vi "FlexMag - 23-03-2023.vi"() -> ()   [LabVIEW 2018] (continued)
                  }
                  frame #1 {
                    n264 = Wait (ms)(milliseconds to wait=u32 500) -> ()  [unwired: 1 out]
                  }
                  frame #2 {
                    n265 = local write "CH3_MP_DO"(TRUE ("CH3_MP_DO")) -> ()
                  }
                }
              }
            }
          }
        }
        n266 = case shown="True" w560 {
          tunnel: "mp3 stop safety" -> [_ w668]
          frame False {
          }
          frame True {
            n267 = case shown="True" w668 {
              frame False {
                n268 = local write "Warning Message"("CH3 MP Cannot be stopped !" ("Warning Message")) -> ()
              }
              frame True {
                n269 = stacked-sequence {
                  frame #0 {
                    w670 = FALSE ("CH3_MP_DO")
                    n270 = local write "CH3_MP_DO"(w670) -> ()
                    n271 = local write "CH3_PL_ATM_DO"(w670) -> ()
                    n272 = local write "CH3_CH_ATM_DO"(w670) -> ()
                  }
                  frame #1 {
                    n273 = Wait (ms)(milliseconds to wait=u32 500) -> ()  [unwired: 1 out]
                  }
                  frame #2 {
                    n274 = local write "CH3_PL_VBV_DO"(TRUE ("CH3_PL_VBV_DO")) -> ()
                  }
                }
              }
            }
          }
        }
        n275 = case shown="True" w562 {
          tunnel: "mp4 start safety" -> [_ w663]
          frame False {
          }
          frame True {
            n276 = case shown="True" w663 {
              frame False {
                n277 = local write "Warning Message"("CH4 MP Cannot be started !" ("Warning Message")) -> ()
              }
              frame True {
                n278 = stacked-sequence {
                  frame #0 {
                    w665 = TRUE ("CH1_PL_ATM_DO")
                    n279 = local write "CH4_PL_ATM_DO"(w665) -> ()
                    n280 = local write "CH4_CH_ATM_DO"(w665) -> ()
                  }
                  frame #1 {
                    n281 = Wait (ms)(milliseconds to wait=u32 500) -> ()  [unwired: 1 out]
                  }
                  frame #2 {
                    n282 = local write "CH4_MP_DO"(TRUE ("CH4_MP_DO")) -> ()
                  }
                }
              }
            }
          }
        }
        n283 = case shown="True" w561 {
          tunnel: "mp4 stop safety" -> [_ w658]
          frame False {
          }
          frame True {
            n284 = case shown="True" w658 {
              frame False {
                n285 = local write "Warning Message"("CH4 MP Cannot be stopped !" ("Warning Message")) -> ()
              }
              frame True {
                n286 = stacked-sequence {
                  frame #0 {
                    w660 = FALSE ("CH4_MP_DO")
                    n287 = local write "CH4_MP_DO"(w660) -> ()
                    n288 = local write "CH4_PL_ATM_DO"(w660) -> ()
                    n289 = local write "CH4_CH_ATM_DO"(w660) -> ()
                  }
                  frame #1 {
                    n290 = Wait (ms)(milliseconds to wait=u32 500) -> ()  [unwired: 1 out]
                  }
                  frame #2 {
                    n291 = local write "CH4_PL_VBV_DO"(TRUE ("CH4_PL_VBV_DO")) -> ()
                  }
                }
              }
            }
          }
        }
        n292 = case shown="True" w503 {
          tunnel: "tpbv1 open safety" -> [_ w640]
          frame False {
          }
          frame True {
            n293 = case shown="True" w640 {
              frame False {
                n294 = local write "Warning Message"("CH1 TP BV Cannot be opened !" ("Warning Message")) -> ()
              }
              frame True {
                n295 = local write "CH1_TP_BV_DO"(TRUE ("CH1_MP_DO")) -> ()
              }
            }
          }
        }
        n296 = case shown="True" w504 {
          tunnel: "tpbv1 close safety" -> [_ w637]
          frame False {
          }
          frame True {
            n297 = case shown="True" w637 {
              frame False {
                n298 = local write "Warning Message"("CH1 TP BV Cannot be closed !" ("Warning Message")) -> ()
              }
              frame True {
                n299 = local write "CH1_TP_BV_DO"(FALSE ("CH1_MP_DO")) -> ()
              }
            }
          }
        }
        n300 = case shown="True" w506 {
          tunnel: "tpbv2 open safety" -> [_ w634]
          frame False {
          }
          frame True {
            n301 = case shown="True" w634 {
              frame False {
                n302 = local write "Warning Message"("CH2 TP BV Cannot be opened !" ("Warning Message")) -> ()
              }
              frame True {
                n303 = local write "CH2_TP_BV_DO"(TRUE ("CH2_MP_DO")) -> ()
              }
            }
          }
        }
        n304 = case shown="True" w505 {
          tunnel: "tpbv2 close safety" -> [_ w631]
          frame False {
          }
          frame True {
            n305 = case shown="True" w631 {
              frame False {
                n306 = local write "Warning Message"("CH2 TP BV Cannot be closed !" ("Warning Message")) -> ()
              }
              frame True {
                n307 = local write "CH2_TP_BV_DO"(FALSE ("CH2_MP_DO")) -> ()
              }
            }
          }
        }
        n308 = case shown="True" w510 {
          tunnel: "tpbv3 open safety" -> [_ w628]
          frame False {
          }
          frame True {
            n309 = case shown="True" w628 {
              frame False {
                n310 = local write "Warning Message"("CH3 TP BV Cannot be opened !" ("Warning Message")) -> ()
              }
              frame True {
                n311 = local write "CH3_TP_BV_DO"(TRUE ("CH3_MP_DO")) -> ()
              }
            }
          }
        }
        n312 = case shown="True" w509 {
          tunnel: "tpbv3 close safety" -> [_ w625]
          frame False {
          }
          frame True {
            n313 = case shown="True" w625 {
              frame False {
                n314 = local write "Warning Message"("CH3 TP BV Cannot be closed !" ("Warning Message")) -> ()
              }
              frame True {
                n315 = local write "CH3_TP_BV_DO"(FALSE ("CH3_MP_DO")) -> ()
              }
            }
          }
        }
        n316 = case shown="True" w507 {
          tunnel: "tpbv4 open safety" -> [_ w622]
          frame False {
          }
          frame True {
            n317 = case shown="True" w622 {
              frame False {
                n318 = local write "Warning Message"("CH4 TP BV Cannot be opened !" ("Warning Message")) -> ()
              }
              frame True {
                n319 = local write "CH4_TP_BV_DO"(TRUE ("CH4_MP_DO")) -> ()
              }
            }
          }
        }
        n320 = case shown="True" w508 {
          tunnel: "tpbv4 close safety" -> [_ w619]
          frame False {
          }
          frame True {
            n321 = case shown="True" w619 {
              frame False {
                n322 = local write "Warning Message"("CH4 TP BV Cannot be closed !" ("Warning Message")) -> ()
              }
              frame True {
                n323 = local write "CH4_TP_BV_DO"(FALSE ("CH4_MP_DO")) -> ()
              }
            }
          }
        }
        n324 = Or(x="plvbv1 open gui", y="plvbv1 open gui 1") -> (x .or. y?=w511:bool)
        n325 = Or(x="plvbv2 open gui", y="plvbv2 open gui 1") -> (x .or. y?=w516:bool)
        n326 = Or(x="plvbv3 open gui", y="plvbv3 open gui 1") -> (x .or. y?=w522:bool)
        n327 = Or(x="plvbv4 open gui", y="plvbv4 open gui 1") -> (x .or. y?=w519:bool)
        n328 = Or(x="chvbv1 open gui", y="chvbv1 open gui 1") -> (x .or. y?=w478:bool)
        n329 = Or(x="chvbv2 open gui", y="chvbv2 open gui 1") -> (x .or. y?=w475:bool)
        n330 = Or(x="chvbv3 open gui", y="chvbv3 open gui 1") -> (x .or. y?=w471:bool)
        n331 = Or(x="chvbv4 open gui", y="chvbv4 open gui 1") -> (x .or. y?=w474:bool)
        n332 = Or(x="plvbv1 close gui", y="plvbv1 close gui 1") -> (x .or. y?=w513:bool)
        n333 = Or(x="plvbv2 close gui", y="plvbv2 close gui 1") -> (x .or. y?=w515:bool)
        n334 = Or(x="plvbv3 close gui", y="plvbv3 close gui 1") -> (x .or. y?=w521:bool)
        n335 = Or(x="plvbv4 close gui", y="plvbv4 close gui 1") -> (x .or. y?=w520:bool)
        n336 = Or(x="chvbv1 close gui", y="chvbv1 close gui 1") -> (x .or. y?=w477:bool)
        n337 = Or(x="chvbv2 close gui", y="chvbv2 close gui 1") -> (x .or. y?=w476:bool)
        n338 = Or(x="chvbv3 close gui", y="chvbv3 close gui 1") -> (x .or. y?=w472:bool)
        n339 = Or(x="chvbv4 close gui", y="chvbv4 close gui 1") -> (x .or. y?=w473:bool)
        n340 = Compound Arithmetic op=OR("bgbv1 open gui 2", "bgbv1 open gui", "bgbv1 open gui 3") -> (w440:bool)
        n341 = Compound Arithmetic op=OR("bgbv2 open gui 2", "bgbv2 open gui", "bgbv1 open gui 1") -> (w443:bool)
        n342 = Compound Arithmetic op=OR("bgbv3 open gui 2", "bgbv3 open gui", "bgbv3 open gui 1") -> (w447:bool)
        n343 = Compound Arithmetic op=OR("bgbv4 open gui 2", "bgbv4 open gui", "bgbv4 open gui 1") -> (w444:bool)
        n344 = Compound Arithmetic op=OR("bgbv1 close gui 2", "bgbv1 close gui", "bgbv1 close gui 1") -> (w441:bool)
        n345 = Compound Arithmetic op=OR("bgbv2 close gui 2", "bgbv2 close gui", "bgbv2 close gui 1") -> (w442:bool)
        n346 = Compound Arithmetic op=OR("bgbv3 close gui 2", "bgbv3 close gui", "bgbv3 close gui 1") -> (w446:bool)
        n347 = Compound Arithmetic op=OR("bgbv4 close gui 2", "bgbv4 close gui", "bgbv4 close gui 1") -> (w445:bool)
        n348 = case shown="True" w511 {
          tunnel: "plvbv1 open safety" -> [_ w656]
          frame False {
          }
          frame True {
            n349 = case shown="True" w656 {
              frame False {
                n350 = local write "Warning Message"("CH1 PL VBV Cannot be opened !" ("Warning Message")) -> ()
              }
              frame True {
              }
            }
          }
        }
        n351 = case shown="True" w513 {
          frame False {
          }
          frame True {
            n352 = local write "CH1_PL_VBV_DO"(FALSE ("CH1_PL_VBV_DO")) -> ()
          }
        }
        n353 = case shown="True" w516 {
          tunnel: "plvbv2 open safety" -> [_ w652]
          frame False {
          }
          frame True {
            n354 = case shown="True" w652 {
              frame False {
                n355 = local write "Warning Message"("CH2 PL VBV Cannot be opened !" ("Warning Message")) -> ()
              }
              frame True {
                n356 = local write "CH2_PL_VBV_DO"(TRUE ("CH2_PL_VBV_DO")) -> ()
              }
            }
          }
        }
        n357 = case shown="True" w515 {
          frame False {
          }
          frame True {
            n358 = local write "CH2_PL_VBV_DO"(FALSE ("CH2_PL_VBV_DO")) -> ()
          }
        }
        n359 = case shown="True" w522 {
          tunnel: "plvbv3 open safety" -> [_ w648]
          frame False {
          }
          frame True {
            n360 = case shown="True" w648 {
              frame False {
                n361 = local write "Warning Message"("CH3 PL VBV Cannot be opened !" ("Warning Message")) -> ()
              }
              frame True {
                n362 = local write "CH3_PL_VBV_DO"(TRUE ("CH3_PL_VBV_DO")) -> ()
              }
            }
          }
        }
        n363 = case shown="True" w521 {
          frame False {
          }
          frame True {
            n364 = local write "CH3_PL_VBV_DO"(FALSE ("CH3_PL_VBV_DO")) -> ()
          }
        }
        n365 = case shown="True" w519 {
          tunnel: "plvbv4 open safety" -> [_ w644]
          frame False {
          }
          frame True {
            n366 = case shown="True" w644 {
              frame False {
                n367 = local write "Warning Message"("CH4 PL VBV Cannot be opened !" ("Warning Message")) -> ()
              }
              frame True {
                n368 = local write "CH4_PL_VBV_DO"(TRUE ("CH4_PL_VBV_DO")) -> ()
              }
            }
          }
        }
        n369 = case shown="True" w520 {
          frame False {
          }
          frame True {
            n370 = local write "CH4_PL_VBV_DO"(FALSE ("CH4_PL_VBV_DO")) -> ()
          }
        }
        n371 = case shown="True" w440 {
          tunnel: "bgbv1 open safety" -> [_ w600]
          frame False {
          }
          frame True {
            n372 = case shown="True" w600 {
              frame False {
                n373 = local write "Warning Message"("CH1 BG BV Cannot be opened !" ("Warning Message")) -> ()
              }
              frame True {
                n374 = local write "CH1_BG_BV_DO"(TRUE ("CH1_MP_DO")) -> ()
              }
            }
          }
        }
        n375 = case shown="True" w441 {
          frame False {
          }
          frame True {
            n376 = local write "CH1_BG_BV_DO"(FALSE ("CH1_MP_DO")) -> ()
          }
        }
        n377 = case shown="True" w443 {
          tunnel: "bgbv2 open safety" -> [_ w596]
          frame False {
          }
          frame True {
            n378 = case shown="True" w596 {
              frame False {
                n379 = local write "Warning Message"("CH2 BG BV Cannot be opened !" ("Warning Message")) -> ()
              }
              frame True {
                n380 = local write "CH2_BG_BV_DO"(TRUE ("CH2_MP_DO")) -> ()
              }
            }
          }
        }
        n381 = case shown="True" w442 {
          frame False {
          }
          frame True {
            n382 = local write "CH2_BG_BV_DO"(FALSE ("CH2_MP_DO")) -> ()
          }
        }
        n383 = case shown="True" w447 {
          tunnel: "bgbv3 open safety" -> [_ w592]
          frame False {
          }
          frame True {
            n384 = case shown="True" w592 {
              frame False {
                n385 = local write "Warning Message"("CH3 BG BV Cannot be opened !" ("Warning Message")) -> ()
              }
              frame True {
                n386 = local write "CH3_BG_BV_DO"(TRUE ("CH3_MP_DO")) -> ()
              }
            }
          }
        }
        n387 = case shown="True" w446 {
          frame False {
          }
          frame True {
            n388 = local write "CH3_BG_BV_DO"(FALSE ("CH3_MP_DO")) -> ()
          }
        }
        n389 = case shown="True" w444 {
          tunnel: "bgbv4 open safety" -> [_ w588]
          frame False {
          }
          frame True {
            n390 = case shown="True" w588 {
              frame False {
                n391 = local write "Warning Message"("CH4 BG BV Cannot be opened !" ("Warning Message")) -> ()
              }
              frame True {
                n392 = local write "CH4_BG_BV_DO"(TRUE ("CH4_MP_DO")) -> ()
              }
            }
          }
        }
        n393 = case shown="True" w445 {
          frame False {
          }
          frame True {
            n394 = local write "CH4_BG_BV_DO"(FALSE ("CH4_MP_DO")) -> ()
          }
        }
        n395 = case shown="True" w478 {
          tunnel: "chvbv1 open safety" -> [_ w616]
          frame False {
          }
          frame True {
            n396 = case shown="True" w616 {
              frame False {
                n397 = local write "Warning Message"("CH1 VBV Cannot be opened !" ("Warning Message")) -> ()
              }
              frame True {
                n398 = local write "CH1_CH_VBV_DO"(TRUE ("CH1_MP_DO")) -> ()
              }
            }
          }
        }
        n399 = case shown="True" w477 {
          frame False {
          }
          frame True {
            n400 = local write "CH1_CH_VBV_DO"(FALSE ("CH1_MP_DO")) -> ()
          }
        }
        n401 = case shown="True" w475 {
          tunnel: "chvbv2 open safety" -> [_ w612]
          frame False {
          }
          frame True {
            n402 = case shown="True" w612 {
              frame False {
                n403 = local write "Warning Message"("CH2 VBV Cannot be opened !" ("Warning Message")) -> ()
              }
              frame True {
                n404 = local write "CH2_CH_VBV_DO"(TRUE ("CH2_MP_DO")) -> ()
              }
            }
          }
        }
        n405 = case shown="True" w476 {
          frame False {
          }
          frame True {
            n406 = local write "CH2_CH_VBV_DO"(FALSE ("CH2_MP_DO")) -> ()
          }
        }
        n407 = case shown="True" w471 {
          tunnel: "chvbv3 open safety" -> [_ w608]
          frame False {
          }
          frame True {
            n408 = case shown="True" w608 {
              frame False {
                n409 = local write "Warning Message"("CH3 VBV Cannot be opened !" ("Warning Message")) -> ()
              }
              frame True {
                n410 = local write "CH3_CH_VBV_DO"(TRUE ("CH3_MP_DO")) -> ()
              }
            }
          }
        }
        n411 = case shown="True" w472 {
          frame False {
          }
          frame True {
            n412 = local write "CH3_CH_VBV_DO"(FALSE ("CH3_MP_DO")) -> ()
          }
        }
        n413 = case shown="True" w474 {
          tunnel: "chvbv4 open safety" -> [_ w604]
          frame False {
          }
          frame True {
            n414 = case shown="True" w604 {
              frame False {
                n415 = local write "Warning Message"("CH4 VBV Cannot be opened !" ("Warning Message")) -> ()
              }
              frame True {
                n416 = local write "CH4_CH_VBV_DO"(TRUE ("CH4_MP_DO")) -> ()
              }
            }
          }
        }
        n417 = case shown="True" w473 {
          frame False {
          }
          frame True {
            n418 = local write "CH4_CH_VBV_DO"(FALSE ("CH4_MP_DO")) -> ()
          }
        }
      }
      frame #1 {
        n419 = Or(x="ch1 trnsbp left open gui", y="ch1 trnsbp left open gui1") -> (x .or. y?=w791:bool)
        n420 = Or(x="ch2 trnsbp right open gui", y="ch2 trnsbp right open gui 1") -> (x .or. y?=w788:bool)
        n421 = Or(x="sov3 open gui", y="sov3 open gui 2") -> (x .or. y?=w801:bool)
        n422 = Or(x="ch2 trnsbp left open gui", y="ch2 trnsbp left open gui 1") -> (x .or. y?=w781:bool)
        n423 = Or(x="ch1 trnsbp left close gui", y="ch1 trnsbp left close gui 1") -> (x .or. y?=w793:bool)
        n424 = Or(x="ch2 trnsbp right close gui", y="ch2 trnsbp right close gui 1") -> (x .or. y?=w787:bool)
        n425 = Or(x="ch3 trnsbp right open gui", y="ch3 trnsbp right open gui 1") -> (x .or. y?=w775:bool)
        n426 = Or(x="sov1 open gui", y="sov1 open gui 2") -> (x .or. y?=w823:bool)
        n427 = Or(x="sov3 close gui", y="sov3 close gui 2") -> (x .or. y?=w802:bool)
        n428 = Or(x="ch2 trnsbp left close gui", y="ch2 trnsbp left close gui 1") -> (x .or. y?=w782:bool)
        n429 = Or(x="ch3 trnsbp left open gui", y="ch3 trnsbp left open gui 1") -> (x .or. y?=w767:bool)
        n430 = Or(x="ch4 trnsbp right open gui", y="ch4 trnsbp right open gui 1") -> (x .or. y?=w762:bool)
        n431 = Or(x="ch3 trnsbp right close gui", y="ch3 trnsbp right close gui 1") -> (x .or. y?=w774:bool)
        n432 = Or(x="sov1 close gui", y="sov1 close gui 2") -> (x .or. y?=w820:bool)
        n433 = Or(x="ch3 trnsbp left close gui", y="ch3 trnsbp left close gui 1") -> (x .or. y?=w768:bool)
        n434 = Or(x="ch4 trnsbp right close gui", y="ch4 trnsbp right close gui 1") -> (x .or. y?=w761:bool)
        n435 = case shown="True" w788 {
          tunnel: "ch2 trnsbp right open safety" -> [_ w908]
          frame False {
          }
          frame True {
            n436 = case shown="True" w908 {
              frame False {
                n437 = local write "Warning Message"("CH2 TRNS BP Right Cannot be opened !" ("Warning Message")) -> ()
              }
              frame True {
                n438 = local write "CH2_Trns_BP_Right_DO"(TRUE ("CH4_MP_DO")) -> ()
              }
            }
          }
        }
        n439 = case shown="True" w781 {
          tunnel: "ch2 trnsbp left open safety" -> [_ w904]
          frame False {
          }
          frame True {
            n440 = case shown="True" w904 {
              frame False {
                n441 = local write "Warning Message"("CH2 TRNS BP Left Cannot be opened !" ("Warning Message")) -> ()
              }
              frame True {
                n442 = local write "CH2_Trns_BP_Left_DO"(TRUE ("CH4_MP_DO")) -> ()
              }
            }
          }
        }
        n443 = case shown="True" w793 {
          frame False {
          }
          frame True {
            n444 = local write "CH1_Trns_BP_Left_DO"(FALSE ("CH4_MP_DO")) -> ()
          }
        }
        n445 = case shown="True" w787 {
          frame False {
          }
          frame True {
            n446 = local write "CH2_Trns_BP_Right_DO"(FALSE ("CH4_MP_DO")) -> ()
          }
        }
        n447 = case shown="True" w775 {
          tunnel: "ch3 trnsbp right open safety" -> [_ w900]
          frame False {
          }
          frame True {
            n448 = case shown="True" w900 {
              frame False {
                n449 = local write "Warning Message"("CH3 TRNS BP Right Cannot be opened !" ("Warning Message")) -> ()
              }
              frame True {
                n450 = local write "CH3_Trns_BP_Right_DO"(TRUE ("CH4_MP_DO")) -> ()
              }
            }
          }
        }
        n451 = case shown="True" w802 {
          frame False {
          }
          frame True {
            n452 = local write "CH3_SoV_Ar_DO"(FALSE ("CH4_MP_DO")) -> ()
          }
        }
        n453 = case shown="True" w782 {
          frame False {
          }
          frame True {
            n454 = local write "CH2_Trns_BP_Left_DO"(FALSE ("CH4_MP_DO")) -> ()
          }
        }
        n455 = case shown="True" w767 {
          tunnel: "ch3 trnsbp left open safety" -> [_ w896]
          frame False {
          }
          frame True {
            n456 = case shown="True" w896 {
              frame False {
                n457 = local write "Warning Message"("CH3 TRNS BP Left Cannot be opened !" ("Warning Message")) -> ()
              }
              frame True {
                n458 = local write "CH3_Trns_BP_Left_DO"(TRUE ("CH4_MP_DO")) -> ()
              }
            }
          }
        }
        n459 = case shown="True" w762 {
          tunnel: "ch4 trnsbp right open safety" -> [_ w892]
          frame False {
          }
          frame True {
            n460 = case shown="True" w892 {
              frame False {
                n461 = local write "Warning Message"("CH4 TRNS BP Right Cannot be opened !" ("Warning Message")) -> ()
              }
              frame True {
                n462 = local write "CH4_Trns_BP_Right_DO"(TRUE ("CH4_MP_DO")) -> ()
              }
            }
          }
        }
        n463 = case shown="True" "CH1 petcool up" {
          frame False {
          }
          frame True {
            n464 = local write "CH1_PetCool_Down_DO"(FALSE ("CH4_MP_DO")) -> ()
            n465 = local write "CH1_PetCool_Up_DO"(TRUE ("CH4_MP_DO")) -> ()
          }
        }
        n466 = case shown="True" "CH2 petcool up" {
          frame False {
          }
          frame True {
            n467 = local write "CH2_PetCool_Down_DO"(FALSE ("CH4_MP_DO")) -> ()
            n468 = local write "CH2_PetCool_Up_DO"(TRUE ("CH4_MP_DO")) -> ()
          }
        }
        n469 = case shown="True" w791 {
          tunnel: "ch1 trnsbp left open safety" -> [_ w912]
          frame False {
          }
          frame True {
            n470 = case shown="True" w912 {
              frame False {
                n471 = local write "Warning Message"("CH1 TRNS BP Left Cannot be opened !" ("Warning Message")) -> ()
              }
              frame True {
                n472 = local write "CH1_Trns_BP_Left_DO"(TRUE ("CH4_MP_DO")) -> ()
              }
            }
          }
        }
        n473 = case shown="True" w774 {
          frame False {
          }
          frame True {
            n474 = local write "CH3_Trns_BP_Right_DO"(FALSE ("CH4_MP_DO")) -> ()
          }
        }
        n475 = case shown="True" "CH1 petcool down" {
          frame False {
          }
          frame True {
            n476 = local write "CH1_PetCool_Down_DO"(TRUE ("CH4_MP_DO")) -> ()
            n477 = local write "CH1_PetCool_Up_DO"(FALSE ("CH4_MP_DO")) -> ()
          }
        }
        n478 = case shown="True" "CH2 petcool down" {
          frame False {
          }
          frame True {
            n479 = local write "CH2_PetCool_Down_DO"(TRUE ("CH4_MP_DO")) -> ()
            n480 = local write "CH2_PetCool_Up_DO"(FALSE ("CH4_MP_DO")) -> ()
          }
        }
        n481 = case shown="True" w820 {
          frame False {
          }
          frame True {
            n482 = local write "CH1_SoV_Ar_DO"(FALSE ("CH4_MP_DO")) -> ()
          }
        }
        n483 = case shown="True" w801 {
          tunnel: "sov3 open safety" -> [_ w916]
          frame False {
          }
          frame True {
            n484 = case shown="True" w916 {
              frame False {
                n485 = local write "Warning Message"("CH3 SoV Ar Cannot be opened !" ("Warning Message")) -> ()
              }
              frame True {
                n486 = local write "CH3_SoV_Ar_DO"(TRUE ("CH4_MP_DO")) -> ()
              }
            }
          }
        }
        n487 = case shown="True" w768 {
          frame False {
          }
          frame True {
            n488 = local write "CH3_Trns_BP_Left_DO"(FALSE ("CH4_MP_DO")) -> ()
          }
        }
        n489 = case shown="True" w761 {
          frame False {
          }
          frame True {
            n490 = local write "CH4_Trns_BP_Right_DO"(FALSE ("CH4_MP_DO")) -> ()
          }
        }
        n491 = case shown="True" "CH3 petcool up" {
          frame False {
          }
          frame True {
            n492 = local write "CH3_PetCool_Down_DO"(FALSE ("CH4_MP_DO")) -> ()
            n493 = local write "CH3_PetCool_Up_DO"(TRUE ("CH4_MP_DO")) -> ()
          }
        }
        n494 = case shown="True" "CH4 petcool up" {
          frame False {
          }
          frame True {
            n495 = local write "CH4_PetCool_Down_DO"(FALSE ("CH4_MP_DO")) -> ()
            n496 = local write "CH4_PetCool_Up_DO"(TRUE ("CH4_MP_DO")) -> ()
          }
        }
        n497 = case shown="True" "ch3 mag active gui" {
          frame False {
          }
          frame True {
            n498 = local write "DCPS_ SW1 DO"(FALSE ("CH4_MP_DO")) -> ()
            n499 = local write "DCPS_ SW2 DO"(TRUE ("CH4_MP_DO")) -> ()
          }
        }
        n500 = case shown="True" "ch2 mag active gui" {
          frame False {
          }
          frame True {
            n501 = local write "DCPS_ SW1 DO"(TRUE ("CH4_MP_DO")) -> ()
            n502 = local write "DCPS_ SW2 DO"(FALSE ("CH4_MP_DO")) -> ()
          }
        }
        n503 = case shown="True" "CH3 petcool down" {
          frame False {
          }
          frame True {
            n504 = local write "CH3_PetCool_Down_DO"(TRUE ("CH4_MP_DO")) -> ()
            n505 = local write "CH3_PetCool_Up_DO"(FALSE ("CH4_MP_DO")) -> ()
          }
        }
        n506 = case shown="True" "CH4 petcool down" {
          frame False {
          }
          frame True {
            n507 = local write "CH4_PetCool_Down_DO"(TRUE ("CH4_MP_DO")) -> ()
            n508 = local write "CH4_PetCool_Up_DO"(FALSE ("CH4_MP_DO")) -> ()
          }
        }
        n509 = case shown="True" w823 {
          tunnel: "sov1 open safety" -> [_ w928]
          frame False {
          }
          frame True {
            n510 = case shown="True" w928 {
              frame False {
                n511 = local write "Warning Message"("SoV Ar Cannot be opened !" ("Warning Message")) -> ()
              }
              frame True {
                n512 = local write "CH1_SoV_Ar_DO"(TRUE ("CH4_MP_DO")) -> ()
              }
            }
          }
        }
        n513 = Compound Arithmetic op=OR("CH3-4 trns open gui", "CH3-4 trns close gui 1", "CH3-4 trns open gui 2") -> (w733:bool)
        n514 = Compound Arithmetic op=OR("CH3-4 trns close gui", "CH3-4 trns open gui 1", "CH3-4 trns close gui 2") -> (w732:bool)
        n515 = Or(x="sov4 open gui", y="sov4 open gui 2") -> (x .or. y?=w809:bool)
        n516 = Compound Arithmetic op=OR("CH2-3 trns open gui", "CH2-3 trns open gui 1", "CH2-3 trns open gui 2") -> (w743:bool)
        n517 = Compound Arithmetic op=OR("CH1-2 trns open gui", "CH1-2 trns open gui 2", "CH1-2 trns open gui 1") -> (w749:bool)
        n518 = Or(x="sov2 open gui", y="sov2 open gui 2") -> (x .or. y?=w815:bool)
        n519 = Or(x="sov4 close gui", y="sov4 close gui 2") -> (x .or. y?=w808:bool)
        n520 = Compound Arithmetic op=OR("CH2-3 trns close gui", "CH2-3 trns close gui 1", "CH2-3 trns close gui 2") -> (w742:bool)
        n521 = Compound Arithmetic op=OR("CH1-2 trns close gui", "CH1-2 trns close gui 2", "CH1-2 trns close gui 1") -> (w750:bool)
        n522 = Or(x="sov2 close gui", y="sov2 close gui 2") -> (x .or. y?=w816:bool)
        n523 = case shown="True" "CH4 cstfix up" {
          frame False {
          }
          frame True {
            n524 = local write "CH4_Cst_Fix_DO"(FALSE ("CH4_MP_DO")) -> ()
          }
        }
        n525 = case shown="True" "CH4 cstfix down" {
          frame False {
          }
          frame True {
            n526 = local write "CH4_Cst_Fix_DO"(TRUE ("CH4_MP_DO")) -> ()
          }
        }
        n527 = case shown="True" "CH2 cstfix up" {
          frame False {
          }
          frame True {
            n528 = local write "CH2_Cst_Fix_DO"(FALSE ("CH4_MP_DO")) -> ()
          }
        }
        n529 = case shown="True" "CH2 cstfix down" {
          frame False {
          }
          frame True {
            n530 = local write "CH2_Cst_Fix_DO"(TRUE ("CH4_MP_DO")) -> ()
          }
        }
        n531 = case shown="True" "CH3 cstfix up" {
          frame False {
          }
          frame True {
            n532 = local write "CH3_Cst_Fix_DO"(FALSE ("CH4_MP_DO")) -> ()
          }
        }
        n533 = case shown="True" "CH3 cstfix down" {
          frame False {
          }
          frame True {
            n534 = local write "CH3_Cst_Fix_DO"(TRUE ("CH4_MP_DO")) -> ()
          }
        }
        n535 = case shown="True" "CH1 srv forward" {
          frame False {
          }
          frame True {
            n536 = local write "CH1_SRV1_Piston_Back_DO"(FALSE ("CH4_MP_DO")) -> ()
            n537 = local write "CH1_SRV1_Piston_For_DO"(TRUE ("CH4_MP_DO")) -> ()
          }
        }
        n538 = case shown="True" "CH2 srv forward" {
          frame False {
          }
          frame True {
            n539 = local write "CH2_SRV1_Piston_Back_DO"(FALSE ("CH4_MP_DO")) -> ()
            n540 = local write "CH2_SRV1_Piston_For_DO"(TRUE ("CH4_MP_DO")) -> ()
          }
        }
        n541 = case shown="True" w733 {
          tunnel: "CH3-4 trns open safety" -> [_ w868]
          frame False {
          }
          frame True {
            n542 = case shown="True" w868 {
              frame False {
                n543 = local write "Warning Message"("CH3-CH4 TRNS GV Cannot be opened !" ("Warning Message")) -> ()
              }
              frame True {
                n544 = local write "CH3_Trns_GV_Open_DO"(TRUE ("CH4_MP_DO")) -> ()
                n545 = local write "CH3_Trns_GV_Close_DO"(FALSE ("CH1_Trns_Gv_Close_DO")) -> ()
              }
            }
          }
        }
        n546 = case shown="True" w732 {
          tunnel: "CH3-4 trns close safety" -> [_ w872]
          frame False {
          }
          frame True {
            n547 = case shown="True" w872 {
              frame False {
                n548 = local write "Warning Message"("CH3-CH4 TRNS GV Cannot be closed !" ("Warning Message")) -> ()
              }
              frame True {
                n549 = local write "CH3_Trns_GV_Open_DO"(FALSE ("CH4_MP_DO")) -> ()
                n550 = local write "CH3_Trns_GV_Close_DO"(TRUE ("CH1_Trns_Gv_Close_DO")) -> ()
              }
            }
          }
        }
        n551 = case shown="True" "CH1 cstfix up" {
          frame False {
          }
          frame True {
            n552 = local write "CH1_Cst_Fix_DO"(FALSE ("CH4_MP_DO")) -> ()
          }
        }
        n553 = case shown="True" "CH1 cstfix down" {
          frame False {
          }
          frame True {
            n554 = local write "CH1_Cst_Fix_DO"(TRUE ("CH4_MP_DO")) -> ()
          }
        }
        n555 = case shown="True" "CH1 srv back" {
          frame False {
          }
          frame True {
            n556 = local write "CH1_SRV1_Piston_Back_DO"(TRUE ("CH4_MP_DO")) -> ()
            n557 = local write "CH1_SRV1_Piston_For_DO"(FALSE ("CH4_MP_DO")) -> ()
          }
        }
        n558 = case shown="True" "CH2 srv back" {
          frame False {
          }
          frame True {
            n559 = local write "CH2_SRV1_Piston_Back_DO"(TRUE ("CH4_MP_DO")) -> ()
            n560 = local write "CH2_SRV1_Piston_For_DO"(FALSE ("CH4_MP_DO")) -> ()
          }
        }
        n561 = case shown="True" "CH3 srv forward" {
          frame False {
          }
          frame True {
            n562 = local write "CH3_SRV1_Piston_Back_DO"(FALSE ("CH4_MP_DO")) -> ()
            n563 = local write "CH3_SRV1_Piston_For_DO"(TRUE ("CH4_MP_DO")) -> ()
          }
        }
        n564 = case shown="True" "CH4 srv forward" {
          frame False {
          }
          frame True {
            n565 = local write "CH4_SRV1_Piston_Back_DO"(FALSE ("CH4_MP_DO")) -> ()
            n566 = local write "CH4_SRV1_Piston_For_DO"(TRUE ("CH4_MP_DO")) -> ()
          }
        }
        n567 = case shown="True" "CH3 srv back" {
          frame False {
          }
          frame True {
            n568 = local write "CH3_SRV1_Piston_Back_DO"(TRUE ("CH4_MP_DO")) -> ()
            n569 = local write "CH3_SRV1_Piston_For_DO"(FALSE ("CH4_MP_DO")) -> ()
          }
        }
        n570 = case shown="True" "CH4 srv back" {
          frame False {
          }
          frame True {
            n571 = local write "CH4_SRV1_Piston_Back_DO"(TRUE ("CH4_MP_DO")) -> ()
            n572 = local write "CH4_SRV1_Piston_For_DO"(FALSE ("CH4_MP_DO")) -> ()
          }
        }
        n573 = case shown="True" w743 {
          tunnel: "CH2-3 trns open safety" -> [_ w876]
          frame False {
          }
          frame True {
            n574 = case shown="True" w876 {
              frame False {
                n575 = local write "Warning Message"("CH2-CH3 TRNS GV Cannot be opened !" ("Warning Message")) -> ()
              }
              frame True {
                n576 = local write "CH2_Trns_GV_Open_DO"(TRUE ("CH4_MP_DO")) -> ()
                n577 = local write "CH2_Trns_GV_Close_DO"(FALSE ("CH1_Trns_Gv_Close_DO")) -> ()
              }
            }
          }
        }
        n578 = case shown="True" w742 {
          tunnel: "CH2-3 trns close safety" -> [_ w880]
          frame False {
          }
          frame True {
            n579 = case shown="True" w880 {
              frame False {
                n580 = local write "Warning Message"("CH2-CH3 TRNS GV Cannot be closed !" ("Warning Message")) -> ()
              }
              frame True {
                n581 = local write "CH2_Trns_GV_Open_DO"(FALSE ("CH4_MP_DO")) -> ()
                n582 = local write "CH2_Trns_GV_Close_DO"(TRUE ("CH1_Trns_Gv_Close_DO")) -> ()
              }
            }
          }
        }
        n583 = case shown="True" w749 {
          tunnel: "CH1-2 trns open safety" -> [_ w884]
          frame False {
          }
          frame True {
            n584 = case shown="True" w884 {
              frame False {
                n585 = local write "Warning Message"("CH1-CH2 TRNS GV Cannot be opened !" ("Warning Message")) -> ()
              }
              frame True {
                n586 = local write "CH1_Trns_Gv_Open_DO"(TRUE ("CH4_MP_DO")) -> ()
                n587 = local write "CH1_Trns_Gv_Close_DO"(FALSE ("CH1_Trns_Gv_Close_DO")) -> ()
              }
            }
          }
        }
        n588 = case shown="True" w750 {
          tunnel: "CH1-2 trns close safety" -> [_ w888]
          frame False {
          }
          frame True {
            n589 = case shown="True" w888 {
              frame False {
                n590 = local write "Warning Message"("CH1-CH2 TRNS GV Cannot be closed !" ("Warning Message")) -> ()
              }
              frame True {
                n591 = local write "CH1_Trns_Gv_Open_DO"(FALSE ("CH4_MP_DO")) -> ()
                n592 = local write "CH1_Trns_Gv_Close_DO"(TRUE ("CH1_Trns_Gv_Close_DO")) -> ()
              }
            }
          }
        }
        n593 = case shown="True" w808 {
          frame False {
          }
          frame True {
            n594 = local write "CH4_SoV_Ar_DO"(FALSE ("CH4_MP_DO")) -> ()
          }
        }
        n595 = case shown="True" w816 {
          frame False {
          }
          frame True {
            n596 = local write "CH2_SoV_Ar_DO"(FALSE ("CH4_MP_DO")) -> ()
          }
        }
        n597 = case shown="True" w809 {
          tunnel: "sov4 open safety" -> [_ w920]
          frame False {
          }
          frame True {
            n598 = case shown="True" w920 {
              frame False {
                n599 = local write "Warning Message"("CH4 SoV Ar Cannot be opened !" ("Warning Message")) -> ()
              }
              frame True {
                n600 = local write "CH4_SoV_Ar_DO"(TRUE ("CH4_MP_DO")) -> ()
              }
            }
          }
        }
        n601 = case shown="True" w815 {
          tunnel: "sov2 open safety" -> [_ w924]
          frame False {
          }
          frame True {
            n602 = case shown="True" w924 {
              frame False {
                n603 = local write "Warning Message"("CH3 SoV Ar Cannot be opened !" ("Warning Message")) -> ()
              }
              frame True {
                n604 = local write "CH2_SoV_Ar_DO"(TRUE ("CH4_MP_DO")) -> ()
              }
            }
          }
        }
      }
      frame #2 {
        n605 = case shown="False" "CH2 safety cancel" {
          frame False {
            n606 = local read "CH2_CH_ATM_DI"() -> (w1168:bool)
            n607 = local read "CH2_PL_VBV_DI"() -> (w1234:bool)
            n608 = local read "CH2_PL_ATM_DI"() -> (w1169:bool)
            n609 = local read "CH2_CH_VBV_DI"() -> (w1245:bool)
            n610 = local read "CH2_SoV_Ar_DI"() -> (w1242:bool)
            n611 = local read "Tp2_stop_cmnd"() -> (w1173:bool)
            n612 = local read "ch2 ch pg torr"() -> (w1243:dbl)
            n613 = local read "CH2_TP_BV_DI"() -> (w1217:bool)
            n614 = local read "CH2_MP_DI"() -> (w1238:bool)
            n615 = local read "ch2_3 vacuum level"() -> (w1189:string)
            n616 = Not(x=w1234) -> (.not. x?=w1235:bool)
            n617 = Not(x=w1242) -> (.not. x?=w1241:bool)
            n618 = Not(x=w1245) -> (.not. x?=w1246:bool)
            n619 = Less Or Equal?(x=w1243, y=0.09) -> (x <= y?=w1244:bool)
            n620 = Not(x=w1217) -> (.not. x?=w1216:bool)
            n621 = local read "ch2 ch pg torr"() -> (w1190:dbl)
            n622 = local read "ch2 ch pg torr"() -> (w1191:dbl)
            n623 = Compound Arithmetic op=XOR(w1169, w1168) -> (w1170:bool)
            n624 = Not(x=w1170) -> (.not. x?=w1167:bool)
            n625 = Compound Arithmetic op=AND(w1167, w1235) -> (w1233:bool)
            n626 = Compound Arithmetic op=AND(w1238, w1246, w1244) -> (w1240:bool)
            n627 = Compound Arithmetic op=AND(w1216, w1173) -> (w1215:bool)
            n628 = Compound Arithmetic op=AND(w1240, w1241) -> (w1239:bool)
            n629 = local write "tpbv2 open safety"(w1233) -> ()
            n630 = local write "mp2 stop safety"(w1215) -> ()
            n631 = local write "bgbv2 open safety"(w1240) -> ()
            n632 = Greater Or Equal?(x=w1190, y=0.9) -> (x >= y?=w1192:bool)
            n633 = Equal?(x="ATMOSPHERE" ("y"), y=w1189) -> (x = y?=w1193:bool)
            n634 = Equal?(x=w1189, y="VACUUM") -> (x = y?=w1194:bool)
            n635 = Less Or Equal?(x=w1191, y=0.1) -> (x <= y?=w1195:bool)
            n636 = local write "cc2 open safety"(w1239) -> ()
            n637 = Compound Arithmetic op=AND(w1192, w1193) -> (w1196:bool)
            n638 = Compound Arithmetic op=AND(w1194, w1195) -> (w1197:bool)
            n639 = Or(x=w1196, y=w1197) -> (x .or. y?=w1175:bool)
            n640 = local read "Tp2_stop_cmnd"() -> (w1237:bool)
            n641 = local read "CH2_CH_VBV_DI"() -> (w1211:bool)
            n642 = local read "CH2_PL_VBV_DI"() -> (w1210:bool)
            n643 = local read "CH2_TP_BV_DI"() -> (w1229:bool)
            n644 = local read "CH2_CH_VBV_DI"() -> (w1207:bool)
            n645 = local read "ch2_tp_gui"() -> (w1171:bool)
            n646 = local read "CH2_MP_DI"() -> (w1228:bool)
            n647 = local read "CH2_TP_BV_DI"() -> (w1204:bool)
            n648 = local write "ch2 trnsbp left open safety"(w1175) -> ()
            n649 = local read "ch2 ch pg torr"() -> (w1209:dbl)
            n650 = local read "CH2_MP_DI"() -> (w1203:bool)
            n651 = Not(x=w1171) -> (.not. x?=w1172:bool)
            n652 = Not(x=w1211) -> (.not. x?=w1213:bool)
            n653 = Not(x=w1210) -> (.not. x?=w1212:bool)
            n654 = Not(x=w1229) -> (.not. x?=w1230:bool)
            n655 = Not(x=w1228) -> (.not. x?=w1231:bool)
            n656 = Not(x=w1207) -> (.not. x?=w1206:bool)
            n657 = Less Or Equal?(x=w1209, y=0.7) -> (x <= y?=w1208:bool)
            n658 = Compound Arithmetic op=AND(w1172, w1237) -> (w1236:bool)
            n659 = Compound Arithmetic op=AND(w1212, w1213) -> (w1214:bool)
            n660 = Compound Arithmetic op=AND(w1230, w1231) -> (w1232:bool)
            n661 = Compound Arithmetic op=AND(w1206, w1208, w1204, w1203) -> (w1205:bool)
            n662 = local write "tp2 start safety"(w1205) -> ()
            n663 = local write "tpbv2 close safety"(w1236) -> ()
            n664 = local write "mp2 start safety"(w1214) -> ()
            n665 = local write "plvbv2 open safety"(w1232) -> ()
            n666 = local read "ch1_2 vacuum level"() -> (w1188:string)
            n667 = local read "ch2 ch pg torr"() -> (w1187:dbl)
            n668 = local read "ch2 ch pg torr"() -> (w1186:dbl)
            n669 = local read "CH2_CH_ATM_DI"() -> (w1226:bool)
            n670 = local read "CH2_CH_VBV_DI"() -> (w1224:bool)
            n671 = local read "CH2_Trns_Gv_Close_DI"() -> (w1258:bool)
            n672 = local read "Tp2_stop_cmnd"() -> (w1247:bool)
            n673 = local read "CH2_BG_BV_DI"() -> (w1250:bool)
            n674 = local read "CH2_TP_BV_DI"() -> (w1252:bool)
            n675 = local read "CH2_CC_DI"() -> (w1222:bool)
            n676 = local read "Tp2 speed gui"() -> (w1253:i32)
            n677 = Greater Or Equal?(x=w1187, y=0.9) -> (x >= y?=w1185:bool)
            n678 = Equal?(x="ATMOSPHERE" ("y"), y=w1188) -> (x = y?=w1184:bool)
            n679 = Equal?(x=w1188, y="VACUUM") -> (x = y?=w1183:bool)
            n680 = Less Or Equal?(x=w1186, y=0.1) -> (x <= y?=w1182:bool)
            n681 = local read "CH2_CC_DI"() -> (w1251:bool)
            n682 = local read "CH2_SoV_Ar_DI"() -> (w1219:bool)
            n683 = Compound Arithmetic op=AND(w1185, w1184) -> (w1181:bool)
            n684 = Compound Arithmetic op=AND(w1183, w1182) -> (w1180:bool)
            n685 = Not(x=w1222) -> (.not. x?=w1223:bool)
            n686 = Not(x=w1224) -> (.not. x?=w1225:bool)
            n687 = Not(x=w1226) -> (.not. x?=w1227:bool)
            n688 = Or(x=w1181, y=w1180) -> (x .or. y?=w1174:bool)
            n689 = Less Or Equal?(x=w1253, y=180) -> (x <= y?=w1256:bool)
            n690 = Not(x=w1250) -> (.not. x?=w1249:bool)
            n691 = Not(x=w1251) -> (.not. x?=w1248:bool)
            n692 = Not(x=w1252) -> (.not. x?=w1255:bool)
            n693 = local write "ch2 trnsbp right open safety"(w1174) -> ()
            n694 = Compound Arithmetic op=AND(w1247, w1249, w1248, w1255, w1256, w1258) -> (w1257:bool)
            n695 = Compound Arithmetic op=AND(w1223, w1225, w1227) -> (w1220:bool)
            n696 = local write "chvbv2 open safety"(w1257) -> ()
            n697 = local write "sov2 open safety"(w1220) -> ()
            n698 = Compound Arithmetic op=AND(w1220, w1219) -> (w1221:bool)
            n699 = local write "ch2 mfc set safety"(w1221) -> ()
          }
          frame True {
            w1259 = TRUE ("bgbv2 open safety")
            n700 = local write "bgbv2 open safety"(w1259) -> ()
            n701 = local write "cc2 open safety"(w1259) -> ()
            n702 = local write "tpbv2 open safety"(w1259) -> ()
            n703 = local write "mp2 stop safety"(w1259) -> ()
            n704 = local write "tp2 start safety"(w1259) -> ()
            n705 = local write "tpbv2 close safety"(w1259) -> ()
            n706 = local write "mp2 start safety"(w1259) -> ()
            n707 = local write "plvbv2 open safety"(w1259) -> ()
            n708 = local write "sov2 open safety"(w1259) -> ()
            n709 = local write "ch2 mfc set safety"(w1259) -> ()
            n710 = local write "chvbv2 open safety"(w1259) -> ()
            n711 = local write "ch2 trnsbp right open safety"(w1259) -> ()
            n712 = local write "ch2 trnsbp left open safety"(w1259) -> ()
          }
        }
        n713 = case shown="False" "CH1 safety cancel" {
          frame False {
            n714 = local read "CH1_CH_VBV_DI"() -> (w1334:bool)
            n715 = local read "CH1_SoV_Ar_DI"() -> (w1331:bool)
            n716 = local read "ch1 ch pg torr"() -> (w1337:dbl)
            n717 = local read "CH1_CH_ATM_DI"() -> (w1262:bool)
            n718 = local read "CH1_MP_DI"() -> (w1290:bool)
            n719 = local read "CH1_PL_ATM_DI"() -> (w1263:bool)
            n720 = local read "CH1_PL_VBV_DI"() -> (w1294:bool)
            n721 = local read "Tp1_stop_cmnd"() -> (w1266:bool)
            n722 = local read "CH1_TP_BV_DI"() -> (w1281:bool)
            n723 = local read "ch1_2 vacuum level"() -> (w1268:string)
            n724 = local read "ch1 ch pg torr"() -> (w1269:dbl)
            n725 = local read "ch1 ch pg torr"() -> (w1270:dbl)
            n726 = Not(x=w1334) -> (.not. x?=w1333:bool)
            n727 = Less Or Equal?(x=w1337, y=0.09) -> (x <= y?=w1335:bool)
            n728 = Not(x=w1331) -> (.not. x?=w1330:bool)
            n729 = Not(x=w1294) -> (.not. x?=w1293:bool)
            n730 = Compound Arithmetic op=XOR(w1263, w1262) -> (w1261:bool)
            n731 = Not(x=w1281) -> (.not. x?=w1282:bool)
            n732 = Compound Arithmetic op=AND(w1290, w1333, w1335) -> (w1332:bool)
            n733 = Not(x=w1261) -> (.not. x?=w1260:bool)
            n734 = Compound Arithmetic op=AND(w1260, w1293) -> (w1295:bool)
            n735 = Compound Arithmetic op=AND(w1282, w1266) -> (w1283:bool)
            n736 = Greater Or Equal?(x=w1269, y=0.9) -> (x >= y?=w1271:bool)
            n737 = local write "bgbv1 open safety"(w1332) -> ()
            n738 = Equal?(x="ATMOSPHERE" ("y"), y=w1268) -> (x = y?=w1272:bool)
            n739 = Equal?(x=w1268, y="VACUUM") -> (x = y?=w1273:bool)
            n740 = Less Or Equal?(x=w1270, y=0.1) -> (x <= y?=w1274:bool)
            n741 = Compound Arithmetic op=AND(w1332, w1330) -> (w1329:bool)
            n742 = local write "tpbv1 open safety"(w1295) -> ()
            n743 = local write "mp1 stop safety"(w1283) -> ()
            n744 = local write "cc1 open safety"(w1329) -> ()
            n745 = Compound Arithmetic op=AND(w1271, w1272) -> (w1275:bool)
            n746 = Compound Arithmetic op=AND(w1273, w1274) -> (w1276:bool)
            n747 = Or(x=w1275, y=w1276) -> (x .or. y?=w1267:bool)
            n748 = local write "ch1 trnsbp left open safety"(w1267) -> ()
            n749 = local read "CH1_TP_BV_DI"() -> (w1310:bool)
            n750 = local read "CH1_CH_VBV_DI"() -> (w1328:bool)
            n751 = local read "CH1_TP_BV_DI"() -> (w1323:bool)
            n752 = local read "CH1_MP_DI"() -> (w1311:bool)
            n753 = local read "ch1 ch pg torr"() -> (w1327:dbl)
            n754 = local read "CH1_CH_VBV_DI"() -> (w1287:bool)
            n755 = local read "CH1_PL_VBV_DI"() -> (w1288:bool)
            n756 = local read "Tp1_stop_cmnd"() -> (w1292:bool)
            n757 = local read "CH1_MP_DI"() -> (w1321:bool)
            n758 = local read "ch1_tp_gui"() -> (w1264:bool)
            n759 = Not(x=w1264) -> (.not. x?=w1265:bool)
            n760 = Not(x=w1310) -> (.not. x?=w1309:bool)
            n761 = Not(x=w1311) -> (.not. x?=w1308:bool)
            n762 = Not(x=w1328) -> (.not. x?=w1325:bool)
            n763 = Less Or Equal?(x=w1327, y=0.7) -> (x <= y?=w1324:bool)
            n764 = Not(x=w1287) -> (.not. x?=w1285:bool)
            n765 = Not(x=w1288) -> (.not. x?=w1286:bool)
            n766 = Compound Arithmetic op=AND(w1309, w1308) -> (w1307:bool)
            n767 = Compound Arithmetic op=AND(w1325, w1324, w1323, w1321) -> (w1322:bool)
            n768 = Compound Arithmetic op=AND(w1265, w1292) -> (w1291:bool)
            n769 = Compound Arithmetic op=AND(w1286, w1285) -> (w1284:bool)
            n770 = local write "tp1 start safety"(w1322) -> ()
            n771 = local write "tpbv1 close safety"(w1291) -> ()
            n772 = local write "plvbv1 open safety"(w1307) -> ()
            n773 = local write "mp1 start safety"(w1284) -> ()
            n774 = local read "CH1_CH_ATM_DI"() -> (w1313:bool)
            n775 = local read "CH1_CH_VBV_DI"() -> (w1318:bool)
            n776 = local read "CH1_Trns_Gv_Close_DI"() -> (w1296:bool)
            n777 = local read "CH1_CC_DI"() -> (w1320:bool)
            n778 = local read "Tp1_stop_cmnd"() -> (w1289:bool)
            n779 = local read "CH1_BG_BV_DI"() -> (w1304:bool)
            n780 = local read "CH1_TP_BV_DI"() -> (w1302:bool)
            n781 = local read "Tp1 speed gui"() -> (w1301:i32)
            n782 = local read "CH1_CC_DI"() -> (w1303:bool)
            n783 = local read "CH1_SoV_Ar_DI"() -> (w1312:bool)
            n784 = Not(x=w1320) -> (.not. x?=w1319:bool)
            n785 = Not(x=w1318) -> (.not. x?=w1317:bool)
            n786 = Not(x=w1313) -> (.not. x?=w1316:bool)
            n787 = Less Or Equal?(x=w1301, y=180) -> (x <= y?=w1298:bool)
            n788 = Not(x=w1304) -> (.not. x?=w1305:bool)
            n789 = Not(x=w1303) -> (.not. x?=w1306:bool)
            n790 = Not(x=w1302) -> (.not. x?=w1299:bool)
            n791 = Compound Arithmetic op=AND(w1319, w1317, w1316) -> (w1315:bool)
            n792 = Compound Arithmetic op=AND(w1289, w1305, w1306, w1299, w1298, w1296) -> (w1297:bool)
            n793 = Compound Arithmetic op=AND(w1315, w1312) -> (w1314:bool)
            n794 = local write "sov1 open safety"(w1315) -> ()
            n795 = local write "chvbv1 open safety"(w1297) -> ()
            n796 = local write "ch1 mfc set safety"(w1314) -> ()
          }
          frame True {
            w1338 = TRUE ("bgbv1 open safety")
            n797 = local write "bgbv1 open safety"(w1338) -> ()
            n798 = local write "cc1 open safety"(w1338) -> ()
            n799 = local write "tpbv1 open safety"(w1338) -> ()
            n800 = local write "mp1 stop safety"(w1338) -> ()
            n801 = local write "tp1 start safety"(w1338) -> ()
            n802 = local write "tpbv1 close safety"(w1338) -> ()
            n803 = local write "mp1 start safety"(w1338) -> ()
            n804 = local write "plvbv1 open safety"(w1338) -> ()
            n805 = local write "sov1 open safety"(w1338) -> ()
            n806 = local write "ch1 mfc set safety"(w1338) -> ()
            n807 = local write "chvbv1 open safety"(w1338) -> ()
            n808 = local write "ch1 trnsbp left open safety"(w1338) -> ()
          }
        }
        n809 = case shown="False" "CH3 safety cancel" {
          frame False {
            n810 = local read "CH3_CH_VBV_DI"() -> (w1164:bool)
            n811 = local read "CH3_CH_ATM_DI"() -> (w1075:bool)
            n812 = local read "CH3_PL_ATM_DI"() -> (w1076:bool)
            n813 = local read "CH3_SoV_Ar_DI"() -> (w1159:bool)
            n814 = local read "CH3_PL_VBV_DI"() -> (w1114:bool)
            n815 = local read "Tp3_stop_cmnd"() -> (w1081:bool)
            n816 = local read "ch3 ch pg torr"() -> (w1161:dbl)
            n817 = local read "CH3_TP_BV_DI"() -> (w1110:bool)
            n818 = local read "CH3_MP_DI"() -> (w1133:bool)
            n819 = local read "ch3_4 vacuum level"() -> (w1109:string)
            n820 = local read "ch3 ch pg torr"() -> (w1108:dbl)
            n821 = local read "ch3 ch pg torr"() -> (w1107:dbl)
            n822 = Not(x=w1164) -> (.not. x?=w1165:bool)
            n823 = Less Or Equal?(x=w1161, y=0.09) -> (x <= y?=w1163:bool)
            n824 = Not(x=w1159) -> (.not. x?=w1158:bool)
            n825 = Not(x=w1114) -> (.not. x?=w1113:bool)
            n826 = Not(x=w1110) -> (.not. x?=w1111:bool)
            n827 = Compound Arithmetic op=XOR(w1076, w1075) -> (w1077:bool)
            n828 = Not(x=w1077) -> (.not. x?=w1074:bool)
            n829 = Greater Or Equal?(x=w1108, y=0.9) -> (x >= y?=w1106:bool)
            n830 = Compound Arithmetic op=AND(w1133, w1165, w1163) -> (w1160:bool)
            n831 = Equal?(x="ATMOSPHERE" ("y"), y=w1109) -> (x = y?=w1105:bool)
            n832 = Equal?(x=w1109, y="VACUUM") -> (x = y?=w1104:bool)
            n833 = Less Or Equal?(x=w1107, y=0.1) -> (x <= y?=w1103:bool)
            n834 = Compound Arithmetic op=AND(w1111, w1081) -> (w1112:bool)
            n835 = Compound Arithmetic op=AND(w1160, w1158) -> (w1157:bool)
            n836 = local write "bgbv3 open safety"(w1160) -> ()
            n837 = Compound Arithmetic op=AND(w1074, w1113) -> (w1115:bool)
            n838 = Compound Arithmetic op=AND(w1106, w1105) -> (w1102:bool)
            n839 = Compound Arithmetic op=AND(w1104, w1103) -> (w1101:bool)
            n840 = local write "mp3 stop safety"(w1112) -> ()
            n841 = local write "cc3 open safety"(w1157) -> ()
            n842 = local write "tpbv3 open safety"(w1115) -> ()
            n843 = Or(x=w1102, y=w1101) -> (x .or. y?=w1087:bool)
            n844 = local write "ch3 trnsbp left open safety"(w1087) -> ()
            n845 = local read "CH3_TP_BV_DI"() -> (w1137:bool)
            n846 = local read "CH3_CH_VBV_DI"() -> (w1153:bool)
            n847 = local read "Tp3_stop_cmnd"() -> (w1134:bool)
            n848 = local read "CH3_CH_VBV_DI"() -> (w1129:bool)
            n849 = local read "CH3_TP_BV_DI"() -> (w1151:bool)
            n850 = local read "CH3_MP_DI"() -> (w1136:bool)
            n851 = local read "ch3 ch pg torr"() -> (w1156:dbl)
            n852 = local read "CH3_PL_VBV_DI"() -> (w1128:bool)
            n853 = local read "CH3_MP_DI"() -> (w1079:bool)
            n854 = local read "ch3_tp_gui"() -> (w1078:bool)
            n855 = Not(x=w1153) -> (.not. x?=w1152:bool)
            n856 = Less Or Equal?(x=w1156, y=0.7) -> (x <= y?=w1154:bool)
            n857 = Not(x=w1137) -> (.not. x?=w1138:bool)
            n858 = Not(x=w1136) -> (.not. x?=w1139:bool)
            n859 = Not(x=w1129) -> (.not. x?=w1131:bool)
            n860 = Not(x=w1128) -> (.not. x?=w1130:bool)
            n861 = Not(x=w1078) -> (.not. x?=w1080:bool)
            n862 = Compound Arithmetic op=AND(w1138, w1139) -> (w1140:bool)
            n863 = Compound Arithmetic op=AND(w1152, w1154, w1151, w1079) -> (w1150:bool)
            n864 = Compound Arithmetic op=AND(w1080, w1134) -> (w1135:bool)
            n865 = Compound Arithmetic op=AND(w1130, w1131) -> (w1132:bool)
            n866 = local read "ch2_3 vacuum level"() -> (w1088:string)
            n867 = local write "tp3 start safety"(w1150) -> ()
            n868 = local write "plvbv3 open safety"(w1140) -> ()
            n869 = local write "tpbv3 close safety"(w1135) -> ()
            n870 = local write "mp3 start safety"(w1132) -> ()
            n871 = local read "ch3 ch pg torr"() -> (w1089:dbl)
            n872 = local read "ch3 ch pg torr"() -> (w1090:dbl)
            n873 = Greater Or Equal?(x=w1089, y=0.9) -> (x >= y?=w1091:bool)
            n874 = local read "CH3_CH_ATM_DI"() -> (w1145:bool)
            n875 = Equal?(x="ATMOSPHERE" ("y"), y=w1088) -> (x = y?=w1092:bool)
            n876 = Equal?(x=w1088, y="VACUUM") -> (x = y?=w1093:bool)
            n877 = Less Or Equal?(x=w1090, y=0.1) -> (x <= y?=w1094:bool)
            n878 = local read "CH3_CH_VBV_DI"() -> (w1147:bool)
            n879 = local read "CH3_Trns_Gv_Close_DI"() -> (w1117:bool)